vi "receive_04digital.vi"() -> ()   [LabVIEW 2015]
uses:
  <instrlib>/niUSRP/niUSRP Fetch Rx Data (CDB Cluster).vi
  <vilib>/Waveform/WDTOps.llb/WDT Get Waveform Subset DBL.vi
  Global_bits.vi
panel:
  out "loop":i32
  out "error out 2":errorcluster
  out "bits":i16[](graph)=[1, 1, 1, 0, 0, 1, 1, 0, 0, 0, 1, 0, 0, 1, 1, 0, 0, 1, 0, 0, 1, 1, 1, 0, 0, 0, 1, 1, 1, 0, 0, 0, 0, 1, 0, 0, 1, 1, 1, 0, 0, 1, 0, 0, 1, 1, 0, 0, 1, 0, 0, 1, 0, 0, 1, 1, 0, 0, 0, 0, 0, 0, 0, 0, 0, 0, 0, 0, 0, 0, 0, 0, 0, 0, 0, 0, 0, 0, 0, 0, 0, 0, 0, 0]
  in  "duration":dbl=180.0 format="%#_13g"
  in  "start":i64=570 format="%.3g"
  out "duration samples":dbl format="%.3g"
  out "start samples":dbl format="%.3g"
  out "RN16 Signal":dynamicdata(graph)=[{"t0"=timestamp(3606433766.7684126 s since 1904-01-01), "dt"=1.0, "Y"=[0.175, 0.175, 0.175, 0.175, 0.175, 0.175, 0.175, 0.175, 0.215, 0.215, 0.215, 0.175, 0.175, 0.215, 0.215, 0.175, 0.175, 0.175, 0.215, 0.175, 0.175, 0.215, 0.215, 0.175, 0.175, 0.215, 0.175, 0.175, 0.215, 0.215, 0.215, 0.175, 0.175, 0.175, 0.215, 0.215, 0.215, 0.175, 0.175, 0.175, 0.175, 0.215, 0.175, 0.175, 0.215, 0.215, 0.215, 0.175, 0.175, 0.215, 0.175, 0.175, 0.215, 0.215, 0.175, 0.175, 0.215, 0.175, 0.175, 0.215, 0.175, 0.175, 0.215, 0.215, 0.175, 0.175, 0.175, 0.175, 0.175, 0.175, 0.175, 0.175, 0.175, 0.175, 0.175, 0.175, 0.175, 0.175, 0.175, 0.175, 0.175, 0.175, 0.175, 0.175, 0.175, 0.175, 0.175, 0.175, 0.175, 0.175, 0.175, 0.175, 0.175, 0.175, 0.175, 0.175, 0.175, 0.175, 0.175, 0.175, 0.175, 0.175, 0.175, 0.175, 0.175, 0.175, 0.175, 0.175, 0.175, 0.175, 0.175, 0.175, 0.175, 0.175, 0.175, 0.175, 0.175, 0.175, 0.175, 0.175, 0.175, 0.175, 0.175, 0.175, 0.175, 0.175, 0.175, 0.175, 0.175, 0.175, 0.175, 0.175, 0.175, 0.175, 0.175, 0.175, 0.175, 0.175, 0.175, 0.175, 0.175, 0.175, 0.175, 0.175, 0.175, 0.175, 0.175, 0.175, 0.175, 0.175, 0.175, 0.175, 0.175, 0.175, 0.175, 0.175, 0.175, 0.175, 0.175, 0.175, 0.175, 0.175, 0.175, 0.175, 0.175, 0.175, 0.175, 0.175, 0.175, 0.175, 0.175, 0.175, 0.175, 0.175, 0.175, 0.175, 0.175, 0.175, 0.175, 0.175]}, {"t0"=timestamp(9218730 s since 1904-01-01), "dt"=1.0, "Y"=[0.3406221454373289, 0.34655768196693226, 0.3699121247436734, 0.3517299973790581, 0.3384254947073794, 0.3411404653374814, 0.34074143167382576, 0.3402118928485841, 0.359876376807248, 0.36929015134989673, 0.36851889640970276, 0.3525962561253656, 0.33849434141570145, 0.3654594786702265, 0.3609272999279583, 0.3397710150997326, 0.3409372621460847, 0.343099423997658, 0.3675213137469461, 0.35753253589599227, 0.3380395661773028, 0.3601815709324133, 0.36598654131745245, 0.3401339824154753, 0.3550029907722583, 0.3693381714377156, 0.3424553146988235, 0.3465383513546202, 0.36840782562422997, 0.36895253945912015, 0.3644760369752452, 0.34167471069478295, 0.34122025046570714, 0.33990400073649896, 0.35991311515680935, 0.36943874094531204, 0.3696372340602897, 0.356958581926641, 0.33831755067288294, 0.3419467207624092, 0.342933641646569, 0.36773755709619504, 0.3577537495672942, 0.3393627756521708, 0.36406595467844305, 0.3688571349909874, 0.3694813195422249, 0.35336587588533663, 0.33884031949023713, 0.36495238076583686, 0.3585653979547974, 0.3379657944707438, 0.36027602188610747, 0.3666826025064231, 0.3402621197447257, 0.3501965173870633, 0.369076276295418, 0.34411473745482507, 0.34517841165707935, 0.36978187839052684, 0.35365894486795607, 0.33887154926464585, 0.36461220070966976, 0.36245738489322, 0.3401803193081806, 0.3414144355624166, 0.34092223134430766, 0.3412994711556938, 0.3412114106362285, 0.3412094889632037, 0.3413392349122958, 0.34127968988110113, 0.3413509009247735, 0.3413662512671857, 0.3413467207972696, 0.34133976289972273, 0.3413231506868576, 0.34135551755963184, 0.34133029993144326, 0.3413773502316049, 0.34135929786041513, 0.34134135095000695, 0.34141321477204806, 0.3413776503460844, 0.34125890991623564, 0.34124173560569665, 0.34128987880661327, 0.3412195940033028, 0.34126282365487315, 0.34116428558083095, 0.34128529949055575, 0.3412706182474848, 0.3412036924876057, 0.34128751820142006, 0.3413298742554239, 0.34130402162815104, 0.34138035818525375, 0.3412624524793557, 0.3413346753589862, 0.3413631845280384, 0.34135376586510385, 0.341407573163435, 0.34141730678959614, 0.3414940912243408, 0.34164115272308626, 0.3414583606513532, 0.34155555542771354, 0.3415929649623387, 0.3415089810415655, 0.34164888825056056, 0.34162271215485573, 0.34157517757287764, 0.34169854957308043, 0.34164950572212155, 0.34164014947708876, 0.3416190738145926, 0.341693884420089, 0.3417707824908514, 0.34182911803574995, 0.3417649819089231, 0.34173373310574356, 0.34177695086637133, 0.3419932450668352, 0.34193843767212867, 0.3419384676343426, 0.3419134455474188, 0.34191785301063643, 0.3419732833149206, 0.3418545358996621, 0.3419085204533205, 0.34196691557187636, 0.34202125410156237, 0.3419096073579528, 0.34189282941499166, 0.34198938326208195, 0.3420554963533951, 0.3419917444694633, 0.341909927435726, 0.3420259678905557, 0.34209933368589646, 0.34209157431136594, 0.34207852182959647, 0.34208599153671776, 0.3421127215963964, 0.3421038912154175, 0.34216491923452286, 0.342247075353566, 0.34222189756741567, 0.34223753677883223, 0.3422508594134853, 0.3422200101453592, 0.3423635374657453, 0.34239003911913, 0.3423148636936711, 0.3422895888547122, 0.3424639565210279, 0.3425217226234917, 0.3426236543167105, 0.34234349256159347, 0.3425215866635001, 0.3424507604863647, 0.3424975208947793, 0.34258134947397795, 0.3425437270369512, 0.3428396561246468, 0.3427733519121661, 0.3427545700895519, 0.34273206967624553, 0.3428642031449667, 0.34281332643232065, 0.3426462379592073, 0.3427588784241122, 0.34281078613423044, 0.3426764740060164, 0.34256671154041013, 0.3427075729815847, 0.3426894656626142, 0.3427378634021326, 0.3428201280896649, 0.3427256345037954], "attributes"=variant("NI_ChannelName"=variant(string "Trigger"))}]
  out "Triggered Signal":dynamicdata(graph)=[{"t0"=timestamp(9218160 s since 1904-01-01), "dt"=1.0, "Y"=array[750 elements], "attributes"=variant("NI_ChannelName"=variant(string "Trigger"))}]
  in  "active antenna":string="RX2"
  in  "Channels":string(combo)="0"
  out "Magnitude":cluster{"t0":dbl, "dt":dbl, "Y":dbl[]}(graph)={"t0"=383.45475762, "dt"=5e-07, "Y"=array[2000000 elements]}
  in  "Stop":bool
  out "coerced gain":dbl format="%#_6f"
  out "coerced carrier frequency":dbl=100000.0 format="%#_6p"
  out "coerced IQ rate":dbl=100000.0 format="%#_6p"
  in  "gain":dbl format="%#_6f"
  in  "carrier frequency":dbl=920000000.0 format="%#_6p"
  in  "IQ rate":dbl=2000000.0 format="%#_6p"
  in  "number of samples":i64=2000000
  in  "timeout":dbl=10.0
  out "error out":errorcluster
  in  "device names":refnum<k15>="192.168.10.14"
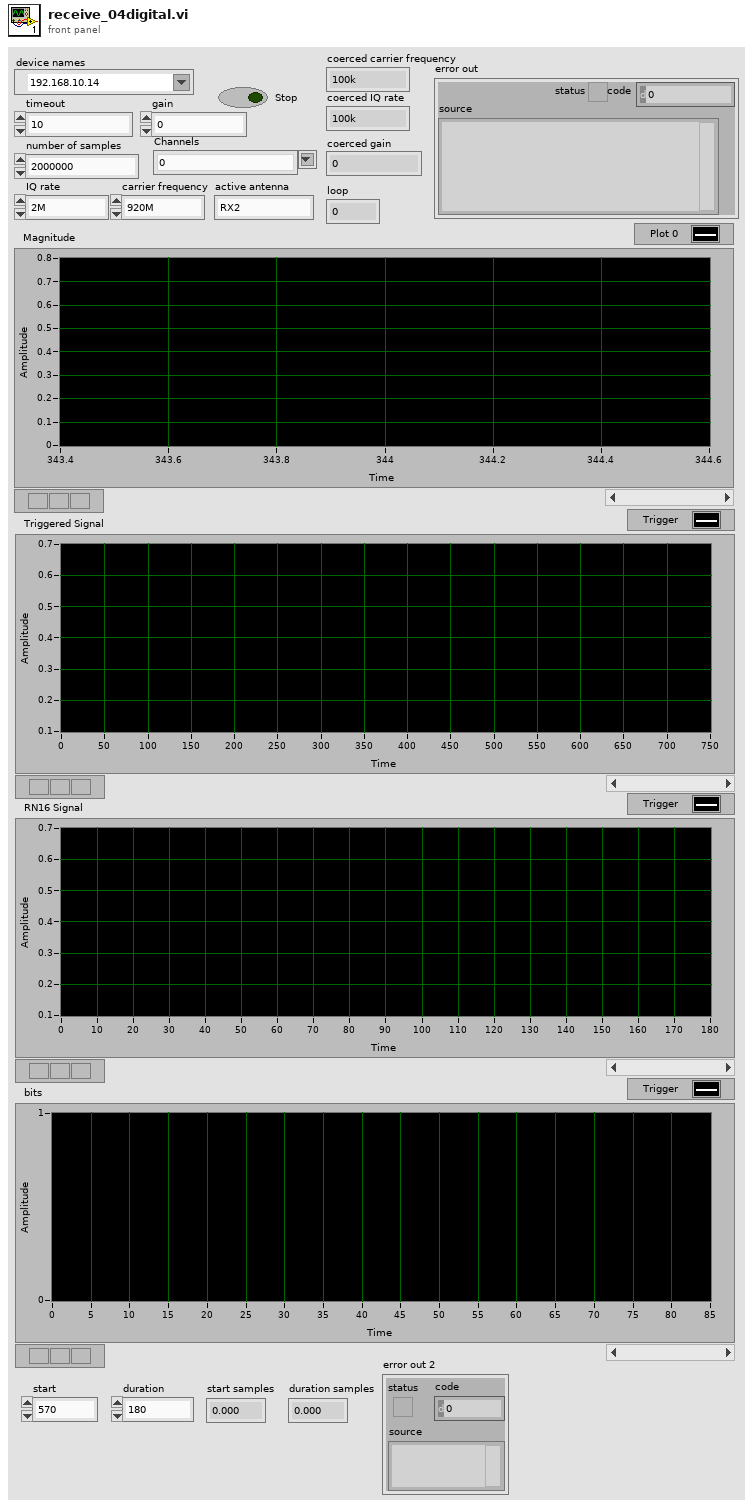
[diagram p1: front panel]
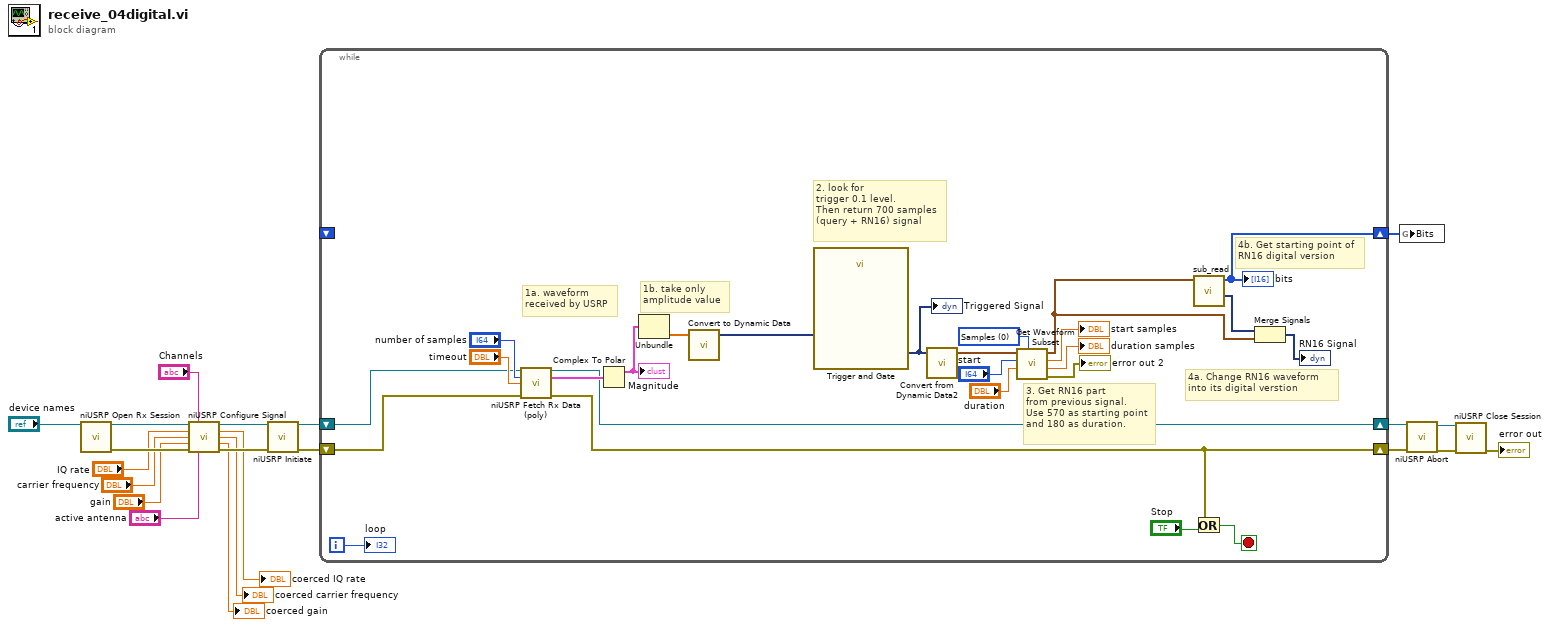
[diagram p0: block diagram]
diagram:
  n1 = call <instrlib>:"niUSRP Open Rx Session.vi"("device names"="device names") -> ("session handle out"=w20:refnum<k15>, "error out"=w19:errorcluster)  [unwired: 13 in]
  n2 = call <instrlib>:"niUSRP Configure Signal.vi"("session handle"=w20, "channel list"="Channels", "IQ rate"="IQ rate", "carrier frequency"="carrier frequency", "gain"="gain", "error in (no error)"=w19, "active antenna"="active antenna") -> ("session handle out"=w18:refnum<k15>, "coerced IQ rate"=→"coerced IQ rate":dbl, "coerced carrier frequency"=→"coerced carrier frequency":dbl, "coerced gain"=→"coerced gain":dbl, "error out"=w17:errorcluster)  [unwired: 4 in]
  n3 = call <instrlib>:"niUSRP Initiate.vi"("session handle"=w18, "error in (no error)"=w17) -> ("session handle out"=w16:refnum<k15>, "error out"=w15:errorcluster)  [unwired: 12 in]
  n4 = while {
    shift-right: [w43] -> w14
    shift-left: w16 -> [w42]
    shift-right: [w25] -> w13
    shift-left: w15 -> [w41]
    shift-right: [w23] -> w1
    shift-left: _ -> [_]
    i -> [w24]
    stop <- w39 stop-if-true
    w36 = u16 0 items=["Samples", "Relative Time"] ("start/duration format")
    # "4b. Get starting point of\nRN16 digital version"
    # "4a. Change RN16 waveform \ninto its digital verstion"
    # "3. Get RN16 part \nfrom previous signal.\nUse 570 as starting point\nand 180 as duration."
    # "2. look for \ntrigger 0.1 level.\nThen return 700 samples\n(query + RN16) signal"
    # "1a. waveform \nreceived by USRP"
    # "1b. take only \namplitude value"
    n5 = call-poly <instrlib>:"niUSRP Fetch Rx Data (poly).vi"("session handle"=w42, "number of samples"="number of samples", "timeout"="timeout", "error in (no error)"=w41) -> ("session handle out"=w43:refnum<k15>, "data"=w44:cluster{"t0":dbl, "dt":dbl, "Y":cdb[]}, "error out"=w25:errorcluster)  [unwired: 8 in, 1 out]
    n6 = Complex To Polar(r * e^(i*theta)=w44) -> (r=w40:cluster{"t0":dbl, "dt":dbl, "Y":dbl[]})  [unwired: 1 out]
    "Magnitude" <- w40
    n7 = Unbundle(w40) -> ("Y"=w28:dbl[])  [unwired: 2 out]
    n8 = call "Convert to Dynamic Data"("Array"=w28) -> ("Dynamic Data Type"=w22:dynamicdata)  [unwired: 3 in]
    n9 = call "Trigger and Gate"("Signals"=w22) -> ("Triggered Signals"=w33:dynamicdata)  [unwired: 7 in, 3 out]
    "Triggered Signal" <- w33
    n10 = call "Convert from Dynamic Data2"("Dynamic Data Type"=w33) -> ("Waveform"=w32:waveform(dbl))  [unwired: 3 in]
    n11 = call-poly <vilib>:"Get Waveform Subset.vi"("start/duration format"=w36, "duration"="duration", "start samples/time"="start", "waveform in"=w32) -> ("error out"=→"error out 2":errorcluster, "actual duration"=→"duration samples":dbl, "actual start samples/time"=→"start samples":dbl, "waveform out"=w29:waveform(dbl))  [unwired: 2 in]
    n12 = call "sub_read.vi"("Raw Signal"=w29) -> ("Digitized Sign"=w31:dynamicdata, "Bits"=w23:i16[])  [unwired: 6 in, 2 out]
    "bits" <- w23
    n13 = Or(x=w25, y="Stop") -> (x .or. y?=w39:bool)
    n14 = Merge Signals(w31, w29) -> (→"RN16 Signal":dynamicdata)
    "loop" <- w24
  }
  n15 = global write "Global_bits.vi" "Bits"(w1) -> ()
  n16 = call <instrlib>:"niUSRP Abort.vi"("session handle"=w14, "error in (no error)"=w13) -> ("session handle out"=w12:refnum<k15>, "error out"=w11:errorcluster)  [unwired: 12 in]
  n17 = call <instrlib>:"niUSRP Close Session.vi"("session handle"=w12, "error in (no error)"=w11) -> ("error out"=→"error out":errorcluster)  [unwired: 13 in]
